vi "Experiment_ANTENNA_GAIN.vi"() -> ()   [LabVIEW 2009]
uses:
  <vilib>/imath/engines/lvmath2/RunTimeEngine/ErrorHandling/NIMS_Finalize Error.vi
  <vilib>/imath/engines/lvmath2/RunTimeEngine/Parser/MC_Version.vi
  <vilib>/imath/engines/lvmath2/RunTimeEngine/Managers/WorkSpace/UID Generator.vi
  <vilib>/imath/engines/lvmath2/RunTimeEngine/NodeEndStatement/NIMS_NodeEndStatement_Output.vi
  <instcachedir>/0/NIMS_NodeEndStatement_Output_B70DDD75627E4997AAE11E9955EDAA25.lvgen/NIMS_NodeEndStatement_Output_B70DDD75627E4997AAE11E9955EDAA25_000.vi
  <vilib>/imath/engines/lvmath2/RunTimeEngine/Managers/SymbolTable/Clear UID.vi
  <vilib>/imath/engines/lvmath/Functions/Error Handling/MergeErrorsWrapper.vi
  <vilib>/imath/engines/lvmath2/RunTimeEngine/LocalVariableDefStatement/MC_LocalVariableDefStatement_Display.vi
  <vilib>/imath/engines/lvmath2/RunTimeEngine/RunTimeType/NIMS_RunTimeType_From StrictType (excl LVString).vi
  <vilib>/imathl/engines/lvmath/Functions/Error Handling/Create Error.vi
  <vilib>/imath/engines/lvmath2/RunTimeEngine/VariableToken/Read/NIMS_Get Elements - RV(_) - Check.vi
  <instcachedir>/0/NIMS_Get Elements - RV(_) - Check_60F12861D0564803969A5D0D0D1716CD.lvgen/NIMS_Get Elements - RV(_) - Check_60F12861D0564803969A5D0D0D1716CD_001.vi
  <instcachedir>/0/NIMS_NodeEndStatement_Output_B70DDD75627E4997AAE11E9955EDAA25.lvgen/NIMS_NodeEndStatement_Output_B70DDD75627E4997AAE11E9955EDAA25_001.vi
  <vilib>/imath/engines/lvmath2/RunTimeEngine/RangeToken/NIMS_Range.vi
  <instcachedir>/0/NIMS_Range_6D647EC16A744C98B5DE1D649A2D648D.lvgen/NIMS_Range_6D647EC16A744C98B5DE1D649A2D648D_001.vi
  <vilib>/imath/engines/lvmath/Functions/Error Handling/error.ctl
  <vilib>/imath/engines/lvmath2/RunTimeEngine/VariableToken/NIMS_VariableToken_CondDefined.vi
  <instcachedir>/0/NIMS_VariableToken_CondDefined_5641E79000FB4D628475532441475385.lvgen/NIMS_VariableToken_CondDefined_5641E79000FB4D628475532441475385_002.vi
  <vilib>/imath/engines/lvmath/Functions/Error Handling/MC_Mask_Errors.vi
  <vilib>/imath/engines/lvmath2/RunTimeEngine/BuiltInFunctions/rem/NIMS_rem_no checks.vi
  <instcachedir>/0/NIMS_rem_no checks_4CC9B305AB7E42EF90AFC4973FB32F8D.lvgen/NIMS_rem_no checks_4CC9B305AB7E42EF90AFC4973FB32F8D_000.vi
  <vilib>/imath/engines/lvmath2/RunTimeEngine/BuiltInFunctions/uint32/NIMS_uint32(real).vi
  <instcachedir>/0/NIMS_uint32(real)_FDC83D68D45943DDB8F3F934FF8A712F.lvgen/NIMS_uint32(real)_FDC83D68D45943DDB8F3F934FF8A712F_000.vi
  <vilib>/imath/engines/lvmath2/RunTimeEngine/BuiltInFunctions/double/NIMS_double.vi
  <instcachedir>/0/NIMS_double_2CE444F3CE4146B199A482FE12545E45.lvgen/NIMS_double_2CE444F3CE4146B199A482FE12545E45_000.vi
  <vilib>/imath/engines/lvmath2/RunTimeEngine/BuiltInFunctions/length/NIMS_length(GV).vi
  <instcachedir>/0/NIMS_length(GV)_7D6E94E728E145E68721C53861296D96.lvgen/NIMS_length(GV)_7D6E94E728E145E68721C53861296D96_000.vi
  <instcachedir>/0/NIMS_Range_6D647EC16A744C98B5DE1D649A2D648D.lvgen/NIMS_Range_6D647EC16A744C98B5DE1D649A2D648D_000.vi
  <vilib>/imath/engines/lvmath2/RunTimeEngine/ReplaceToken/NIMS_Replace - V(S)=S.vi
  <instcachedir>/0/NIMS_Replace - V(S)=S_670A9E0533664C1D848C8E58B3321B6A.lvgen/NIMS_Replace - V(S)=S_670A9E0533664C1D848C8E58B3321B6A_001.vi
  <vilib>/imath/engines/lvmath2/RunTimeEngine/ReplaceToken/NIMS_Replace - Size Check _(_)=S.vi
  <instcachedir>/0/NIMS_Replace - Size Check _(_)=S_8596181D73404097BAB9CBB006194BB0.lvgen/NIMS_Replace - Size Check _(_)=S_8596181D73404097BAB9CBB006194BB0_002.vi
  <vilib>/imath/engines/lvmath2/RunTimeEngine/ReplaceToken/NIMS_Replace - Check Linear.vi
  <instcachedir>/0/NIMS_Replace - Check Linear_9243CBB174894FF6977027453DA6955E.lvgen/NIMS_Replace - Check Linear_9243CBB174894FF6977027453DA6955E_002.vi
  <vilib>/imath/engines/lvmath2/RunTimeEngine/VariableToken/NIMS_VariableToken_CondDefinedDefinedByReplace.vi
  <instcachedir>/0/NIMS_VariableToken_CondDefinedDefinedByReplace_D162CFFC24174562A9FEA619A91E1A56.lvgen/NIMS_VariableToken_CondDefinedDefinedByReplace_D162CFFC24174562A9FEA619A91E1A56_002.vi
  <vilib>/imath/engines/lvmath2/RunTimeEngine/CommandStatement/MC_CommandStatement_break.vi
  <vilib>/imath/engines/lvmath2/RunTimeEngine/ArithmeticOperatorToken/NIMS_ArithmeticOperator_times.vi
  <instcachedir>/0/NIMS_ArithmeticOperator_times_3987BC660D7947CD8628C10658A43225.lvgen/NIMS_ArithmeticOperator_times_3987BC660D7947CD8628C10658A43225_001.vi
  <instcachedir>/0/NIMS_ArithmeticOperator_times_3987BC660D7947CD8628C10658A43225.lvgen/NIMS_ArithmeticOperator_times_3987BC660D7947CD8628C10658A43225_000.vi
  <vilib>/imath/engines/lvmath2/RunTimeEngine/Managers/SymbolTable/NIMS_WorkSpace.lvlib
panel:
  out "error out":errorcluster
  in  "?":enum32{"GAIN MEASUREMENT"}(tab)
  out "?":cluster{"Y":dbl[], "Y":dbl[]}[](graph)
  in  "Samples":i32=3 min=3 max=50 step=1
  out "G":dbl
  out "m":dbl
  in  "HELP FOR GAIN MEASUREMENT":bool
  in  "?":enum32{"ATTENUATOR"}(tab)
  out "?":dbl[](graph)
  in  "Set the value of attenuation in dB":dbl(slide) scale=0.0..100.0
  out "?":errorcluster
  in  "HELP FOR ATTENUATOR":bool
  out "error out":errorcluster
  in  "?":enum32{"ISOLATOR"}(tab)
  out "?":dbl[](graph)
  in  "?":bool
  out "?":errorcluster
  in  "HELP FOR ISOLATOR":bool
  out "error out":errorcluster
  in  "?":enum32{"MODULATOR"}(tab)
  in  "Modulating Frequency(KHz)":dbl(slide) scale=0.5..1.5
  out "?":errorcluster
  out "?":dbl[](graph)
  in  "HELP FOR MODULATOR":bool
  out "error out":errorcluster
  in  "?":enum32{"SOURCE"}(tab)
  out "?":dbl[](graph)
  in  "Frequency of carrier wave(GHz)":dbl(slide) scale=8.0..15.0
  in  "Voltage":dbl(knob) scale=0.0..20.0 scale format="%#_10g"
  out "?":errorcluster
  in  "HELP FOR SOURCE":bool
  out "error out":errorcluster
  # "Source"
  # "Variable Attenuator"
  # "VSWR Meter"
  # "Coaxial to rectangular adapter"
  # "Transmitting and Recieving Antenna"
  # "Isolator"
  # "Connecting Waveguide"
  # "Connecting Waveguide"
  # "Backward Direction"
  # "Forward direction"
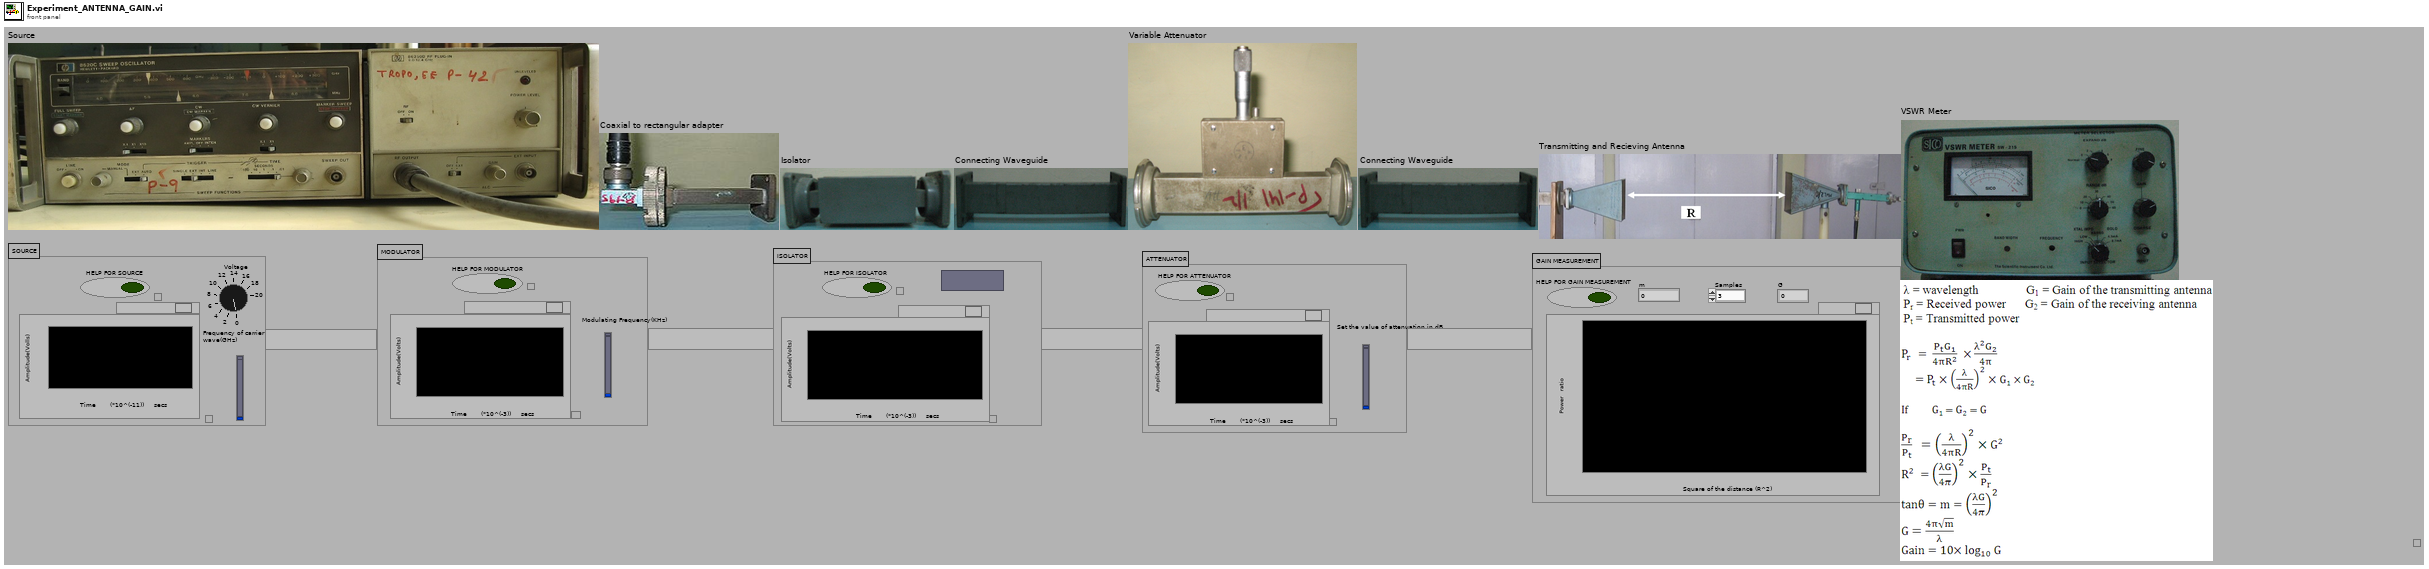
[diagram p1: front panel]
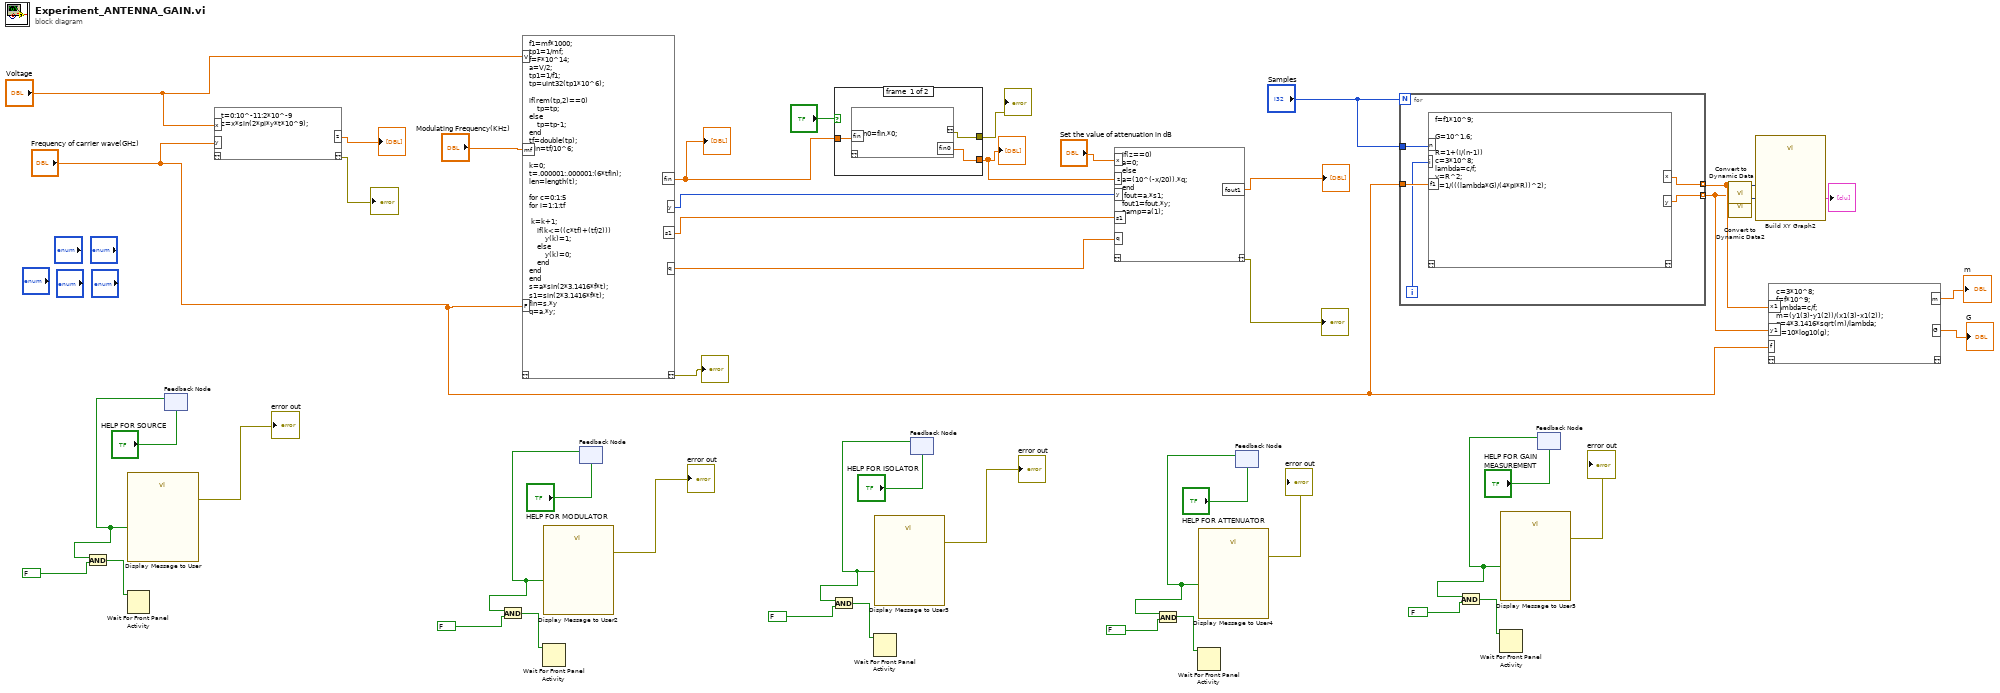
[diagram p0: block diagram]
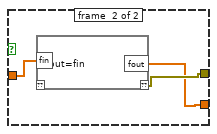
[diagram p2: hidden frame]
diagram:
  n1 = feedback #1("HELP FOR SOURCE") -> (w49:bool)
  n2 = And(x=w49, y=FALSE) -> (x .and. y?=w47:bool)
  n3 = Wait For Front Panel Activity(3:w47) -> ()  [unwired: 3 out]
  n4 = call "Display Message to User"("Enable"=w49) -> ("error out"=→"error out":errorcluster, "CLOSE"=w51:bool)  [unwired: 2 in, 7 out]
  n5 = mathscript code="t=0:10^-11:2*10^-9\nz=x*sin(2*pi*y*t*10^9);"("x"="Voltage", "y"="Frequency of carrier wave(GHz)") -> ("??"=→"?":errorcluster, "z"=→"?":dbl[])  [unwired: 1 in]
  n6 = mathscript code="f1=mf*1000;\ntp1=1/mf;\nf=F*10^14;\na=V/2;\ntp1=1/f1;\ntp=uint32(tp1*10^6);\n\nif(rem(tp,2)==0)\n    tp=tp;\nelse\n    tp=tp-1;\nend\ntf=double(tp);\ntfin=tf/10^6;\n\nk=0;\nt=.000001:.000001:(6*tfin);\nlen=length(t);\n\nfor c=0:1:5\nfor i=1:1:tf\n  \n k=k+1;\n    if(k<=((c*tf)+(tf/2)))\n        y(k)=1;\n    else\n        y(k)=0;\n    end\nend\nend\ns=a*sin(2*3.1416*f*t);\ns1=sin(2*3.1416*f*t);\nfin=s.*y\nq=a.*y;"("V"="Voltage", "mf"="Modulating Frequency(KHz)", "F"="Frequency of carrier wave(GHz)") -> ("??"=→"?":errorcluster, "fin"=w8:dbl[], "y"=w12:i32[], "q"=w13:dbl[], "s1"=w11:dbl[])  [unwired: 1 in]
  "?" <- w8
  n7 = feedback #2("HELP FOR MODULATOR") -> (w43:bool)
  n8 = And(x=w43, y=FALSE) -> (x .and. y?=w41:bool)
  n9 = Wait For Front Panel Activity(3:w41) -> ()  [unwired: 3 out]
  n10 = call "Display Message to User2"("Enable"=w43) -> ("error out"=→"error out":errorcluster, "CLOSE"=w45:bool)  [unwired: 2 in, 7 out]
  n11 = case shown="True" "?" {
    tunnel: w8 -> [w55 w78]
    tunnel: [w57 w77] -> w53
    tunnel: [w56 w76] -> w9
    frame #0 {
      n12 = mathscript code="fin0=fin.*0;"("fin"=w55) -> ("??"=w57:errorcluster, "fin0"=w56:dbl[])  [unwired: 1 in]
    }
    frame #1 {
      n13 = mathscript code="fout=fin"("fin"=w78) -> ("??"=w77:errorcluster, "fout"=w76:dbl[])  [unwired: 1 in]
    }
  }
  "?" <- w9
  "?" <- w53
  n14 = feedback #3("HELP FOR ISOLATOR") -> (w37:bool)
  n15 = And(x=w37, y=FALSE) -> (x .and. y?=w35:bool)
  n16 = Wait For Front Panel Activity(3:w35) -> ()  [unwired: 3 out]
  n17 = call "Display Message to User3"("Enable"=w37) -> ("error out"=→"error out":errorcluster, "CLOSE"=w39:bool)  [unwired: 2 in, 7 out]
  n18 = mathscript code="if(z==0)\na=0;\nelse\na=(10^(-x/20)).*q;\nend\n fout=a.*s1;\nfout1=fout.*y;\nsamp=a(1);"("x"="Set the value of attenuation in dB", "z"=w9, "y"=w12, "s1"=w11, "q"=w13) -> ("??"=→"?":errorcluster, "fout1"=→"?":dbl[])  [unwired: 1 in]
  n19 = feedback #4("HELP FOR ATTENUATOR") -> (w31:bool)
  n20 = And(x=w31, y=FALSE) -> (x .and. y?=w29:bool)
  n21 = Wait For Front Panel Activity(3:w29) -> ()  [unwired: 3 out]
  n22 = call "Display Message to User4"("Enable"=w31) -> ("error out"=→"error out":errorcluster, "CLOSE"=w33:bool)  [unwired: 2 in, 7 out]
  n23 = for {
    N: "Samples" -> [_]
    tunnel: "Frequency of carrier wave(GHz)" -> [w115]
    tunnel: "Samples" -> [w114]
    tunnel: [w113] -> w24 mode=indexing
    tunnel: [w112] -> w21 mode=indexing
    i -> [w111]
    n24 = mathscript code="f=f1*10^9;\n\nG=10^1.6;\n\nR=1+(i/(n-1))\nc=3*10^8;\nlambda=c/f;\ny=R^2;\nx=1/(((lambda*G)/(4*pi*R))^2);"("f1"=w115, "n"=w114, "i"=w111) -> ("y"=w112:dbl, "x"=w113:dbl)  [unwired: 2 out]
  }
  n25 = feedback #5("HELP FOR GAIN MEASUREMENT") -> (w3:bool)
  n26 = And(x=w3, y=FALSE) -> (x .and. y?=w1:bool)
  n27 = Wait For Front Panel Activity(3:w1) -> ()  [unwired: 3 out]
  n28 = call "Display Message to User5"("Enable"=w3) -> ("error out"=→"error out":errorcluster, "CLOSE"=w5:bool)  [unwired: 2 in, 7 out]
  n29 = call "Convert to Dynamic Data"("Array"=w24) -> ("Dynamic Data Type"=w27:dynamicdata)  [unwired: 3 out]
  n30 = call "Convert to Dynamic Data2"("Array"=w21) -> ("Dynamic Data Type"=w26:dynamicdata)  [unwired: 3 out]
  n31 = call "Build XY Graph2"("Y Input"=w26, "X Input"=w27) -> ("XY Graph"=→"?":cluster{"Y":dbl[], "Y":dbl[]}[])  [unwired: 3 in, 6 out]
  n32 = mathscript code="c=3*10^8;\nf=f*10^9;\nlambda=c/f;\nm=(y1(3)-y1(2))/(x1(3)-x1(2));\ng=4*3.1416*sqrt(m)/lambda;\nG=10*log10(g);"("x1"=w24, "y1"=w21, "f"="Frequency of carrier wave(GHz)") -> ("m"=→"m":dbl, "G"=→"G":dbl)  [unwired: 2 out]
